vi "HeartBeatDetectRealTime1Valsalva.vi"() -> ()   [LabVIEW 2014, in "Phonocardiography.lvlib"]
uses:
  Phonocardiography.lvlib
  <vilib>/sound2/lvsound2.llb/Sampling Mode.ctl
  <vilib>/sound2/lvsound2.llb/Sound Data Format.ctl
  <vilib>/Platform/TimedLoop/XDataNode/timing_clust.ctl
  <vilib>/Platform/TimedLoop/XDataNode/nitl_modes.ctl
  <vilib>/Platform/TimedLoop/XDataNode/wakeup.ctl
  <vilib>/sound2/lvsound2.llb/Sound Input Read (DBL).vi
  <vilib>/Waveform/WDTOps.llb/WDT Get Waveform Time Array DBL.vi
  <vilib>/platform/TimedLoop/XDataNode/XDataNode.xnode
  <vilib>/Analysis/NI_AAL_SigProc.lvlib
  <vilib>/Platform/TimedLoop/XDataNode/XDNodeRunTimeDep.lvlib
  <vilib>/Analysis/NI_AALBase.lvlib
panel:
  in  "Exhale length [s]":dbl=6.0
  out "Inhale":bool
  in  "Init length [s]":dbl=6.0
  in  "Stop":bool
  in  "Window length [s]":dbl=0.95 min=0.0 max=50.0 step=0.05
  in  "Save to":path=path "C:/Users/Tamas/Documents/Projektek/Magzati szívhang/Felvételek cikkhez/breath_2.wav"
  in  "Samples per\nLoop":i32=8192
  in  "Device ID":u32
  in  "Stop & Save":bool
  out "Heart rate":T1(graph)=[{"X [s]"=[1.3810454402648886, 2.1451014620294155, 2.834039083155719, 3.5082652214542707, 4.267812415306186, 5.283414824587101, 6.333745411581, 7.352497923020055, 8.340778421797614, 9.286742620731337, 10.168091052124844, 11.008353434253126, 11.766188704199886, 12.459857993882613, 13.160303085008367, 13.937005708439617, 14.916256103906665, 15.990392513713077, 17.026184719534893, 18.025566635405323, 18.97826048371807, 19.895876149785295, 20.77148344893412, 21.58219271330085, 22.317733593752568, 23.026818175608778, 23.777685137270783, 24.65158299378833, 25.66356423384652, 26.69873921266114, 27.752698470400272, 28.772013707647154, 29.742896014934153, 30.650118429443005, 31.470679114349547, 32.19628263399749, 32.89445774972244, 33.66604914709347, 34.53537473985873, 35.51529057371639, 36.547147137879335, 37.577860857157, 38.55405439667892, 39.45290864114518, 40.309631377497524, 41.11504533403093, 41.84509526458157, 42.525847910413134, 43.23209659612331, 44.06765071982923, 44.96984707542182, 45.947480314447624, 46.920868322812716, 47.837254170634964, 48.70405945356165, 49.504490542408455, 50.220753683982565, 50.91447600262699, 51.59735912079533, 52.30215614364477, 53.04693497173172, 53.877926380484645, 54.78308482581491, 55.72546544156374, 56.671367006023424, 57.591099754403, 58.475088172441076, 59.293003678840876, 60.046376669503445, 60.79669511272331, 61.52442997106812, 62.25025157154459, 63.012813377936496, 63.8271252008184, 64.76642444301858, 65.69495143489829, 66.61622522259673, 67.50133872767269, 68.32457083017923, 69.10155513831889, 69.84249179812262, 70.6376427542073, 71.43050342495626, 72.15710097862082, 72.869491186341, 73.59336989453159, 74.37313142224703, 75.27019769563682, 76.15832609501031, 77.03212650593542, 77.90552889801594, 78.77465743537506, 79.62075706292664, 80.45163850714349, 81.1982417174044, 81.8712051082844, 82.52583434169513, 83.20775444122651, 84.0216953422601, 84.87335076971661, 85.79249037575387, 86.73069894059917, 87.64715321189007, 88.53326116001448, 89.36559786895394, 90.15065708658227, 90.87383450984113, 91.54145150844631, 92.21301976186118, 92.94571852487775, 93.7510641244373, 94.64661578749286, 95.54741044208302, 96.5225663414621, 97.52177353097777, 98.48706973490316, 99.44226945816028, 100.37012376206445, 101.23467811616628, 101.98654166591145, 102.67171477694043, 103.36534981417746, 104.11316781035048, 104.97669498014312, 105.91515824719292, 106.88001332870756, 107.80736044827695, 108.70537037239123, 109.55381284940862, 110.3611828413852, 111.11257513889484, 111.80992721929452, 112.53266423876909, 113.371875704155, 114.23971177605979, 115.15354851469199, 116.12435502467058, 117.11297189324033, 118.07091168953183, 118.96774342793292, 119.82781735444664, 120.67884494275361, 121.4691175113743, 122.20823957402418], "Heart Rate [BPM]"=[68.40647655058463, 78.5282731774494, 87.09061337354396, 88.99091357005743, 78.99443311181248, 59.07823716416964, 57.12487167656724, 58.89556033118001, 60.71150859924507, 63.42734753348079, 68.07750245284211, 71.40626699011246, 79.17287882921464, 86.49654942550936, 85.65981939222115, 77.24964251432185, 61.27135641480476, 55.85882710261502, 57.926676473101054, 60.03710798362997, 62.97930873203597, 65.3868522724245, 68.52386915724182, 74.00926896631427, 81.5726244381578, 84.61613964716969, 79.90763086338636, 68.65790956290691, 59.28963663056629, 57.96121547364511, 56.928196758484795, 58.863046295723876, 61.799457616713596, 66.13593209387643, 73.12073452170533, 82.68978633002146, 85.93832499701593, 77.76136463474401, 69.01901945523561, 61.229748440533335, 58.14761671712856, 58.21209020294084, 61.46322175967706, 66.75164563040832, 70.03432668947367, 74.49585335998746, 82.1861594517855, 88.13774043684857, 84.95591031035492, 71.80863369315091, 66.50436972846161, 61.372708705965145, 61.640373093126925, 65.4746034572527, 69.21969810499517, 74.95960718672598, 83.76809655197358, 86.48993752607461, 87.86276656089348, 85.13089308667135, 80.56082925197656, 72.20291253075968, 66.28673721108329, 63.66854219759496, 63.43154748271637, 65.2363418674726, 67.87419243926723, 73.35721053156293, 79.64182515652938, 79.9660471392918, 82.44761029651161, 82.66494130322529, 78.68214680707973, 73.68184805134712, 63.87740701191062, 64.61847692605704, 65.12721929264292, 67.78791607619927, 72.88345512439918, 77.22163674535267, 80.97858191534635, 75.45737012684927, 75.67533895119668, 82.57666117562985, 84.22350468855369, 82.8868142150163, 76.94660209229534, 66.88469044017728, 67.55779912265608, 68.66556624352756, 68.69685787907532, 69.03466797018595, 70.91363480873557, 72.21246835829115, 80.363972690436, 89.15789597639342, 91.65493524844545, 87.98684778646678, 73.71542568239107, 70.45102757014268, 65.27844040872237, 63.951665171478695, 65.46971505243243, 67.71184044449664, 72.0862114521537, 76.42735560925004, 82.96719182634531, 89.87188781195628, 89.34311545387331, 81.88904230297295, 74.50217649765996, 66.99780981399154, 66.60785529116924, 61.528623308544454, 60.047606371890396, 62.1570868672322, 62.81408855040989, 64.66532487647643, 69.39991651806916, 79.80171404816222, 87.56911068779753, 86.50082071834085, 80.23342619066719, 69.48246922492017, 63.93430846645616, 62.18550448613611, 64.70069161142244, 66.81440637661001, 70.71781720656415, 74.31537039555965, 79.85176345147495, 86.03975192217317, 83.01774834174188, 71.49568669490081, 69.13748107785794, 65.6572421128593, 61.80428271059227, 60.69085194429577, 62.6344163091249, 66.9021817927302, 69.7614450925258, 70.5030022814692, 75.92317180478933, 81.17739008478434]}, {"X [s]"=array[1351680 elements], "Heart Rate [BPM]"=array[1351680 elements]}]
  out "pNN50 [%]":dbl=22.377622377622377 format="%0.2f"
  out "rMSSD  [ms]":dbl=63.69905592461299 format="%0.2f"
  out "sdRR [ms]":dbl=107.76134947819452 format="%0.2f"
  out "Mean RR [ms]":dbl=845.1687782348819 format="%0.2f"
  out "Mean heart rate [BPM]":dbl=70.99173744362493
  out "Peaks":cluster{dbl[], "Amplitudes":dbl[]}[](graph)=[{array[1351680 elements], "Amplitudes"=array[1351680 elements]}, {[0.503935508201194, 1.3810454402648886, 2.1451014620294155, 2.834039083155719, 3.5082652214542707, 4.267812415306186, 5.283414824587101, 6.333745411581, 7.352497923020055, 8.340778421797614, 9.286742620731337, 10.168091052124844, 11.008353434253126, 11.766188704199886, 12.459857993882613, 13.160303085008367, 13.937005708439617, 14.916256103906665, 15.990392513713077, 17.026184719534893, 18.025566635405323, 18.97826048371807, 19.895876149785295, 20.77148344893412, 21.58219271330085, 22.317733593752568, 23.026818175608778, 23.777685137270783, 24.65158299378833, 25.66356423384652, 26.69873921266114, 27.752698470400272, 28.772013707647154, 29.742896014934153, 30.650118429443005, 31.470679114349547, 32.19628263399749, 32.89445774972244, 33.66604914709347, 34.53537473985873, 35.51529057371639, 36.547147137879335, 37.577860857157, 38.55405439667892, 39.45290864114518, 40.309631377497524, 41.11504533403093, 41.84509526458157, 42.525847910413134, 43.23209659612331, 44.06765071982923, 44.96984707542182, 45.947480314447624, 46.920868322812716, 47.837254170634964, 48.70405945356165, 49.504490542408455, 50.220753683982565, 50.91447600262699, 51.59735912079533, 52.30215614364477, 53.04693497173172, 53.877926380484645, 54.78308482581491, 55.72546544156374, 56.671367006023424, 57.591099754403, 58.475088172441076, 59.293003678840876, 60.046376669503445, 60.79669511272331, 61.52442997106812, 62.25025157154459, 63.012813377936496, 63.8271252008184, 64.76642444301858, 65.69495143489829, 66.61622522259673, 67.50133872767269, 68.32457083017923, 69.10155513831889, 69.84249179812262, 70.6376427542073, 71.43050342495626, 72.15710097862082, 72.869491186341, 73.59336989453159, 74.37313142224703, 75.27019769563682, 76.15832609501031, 77.03212650593542, 77.90552889801594, 78.77465743537506, 79.62075706292664, 80.45163850714349, 81.1982417174044, 81.8712051082844, 82.52583434169513, 83.20775444122651, 84.0216953422601, 84.87335076971661, 85.79249037575387, 86.73069894059917, 87.64715321189007, 88.53326116001448, 89.36559786895394, 90.15065708658227, 90.87383450984113, 91.54145150844631, 92.21301976186118, 92.94571852487775, 93.7510641244373, 94.64661578749286, 95.54741044208302, 96.5225663414621, 97.52177353097777, 98.48706973490316, 99.44226945816028, 100.37012376206445, 101.23467811616628, 101.98654166591145, 102.67171477694043, 103.36534981417746, 104.11316781035048, 104.97669498014312, 105.91515824719292, 106.88001332870756, 107.80736044827695, 108.70537037239123, 109.55381284940862, 110.3611828413852, 111.11257513889484, 111.80992721929452, 112.53266423876909, 113.371875704155, 114.23971177605979, 115.15354851469199, 116.12435502467058, 117.11297189324033, 118.07091168953183, 118.96774342793292, 119.82781735444664, 120.67884494275361, 121.4691175113743, 122.20823957402418], "Amplitudes"=[0.25504343516715083, 0.26274397594688526, 0.22978339915261922, 0.2925323075507681, 0.2597312409018822, 0.3127614804590793, 0.28443490759254775, 0.27205766410251664, 0.3588946349377459, 0.30343314882440386, 0.31376920698615113, 0.322137223701114, 0.2810882365066251, 0.27506508906369076, 0.30417811837100495, 0.3072988366388709, 0.3531073610883032, 0.35795320527487806, 0.3052941945137585, 0.31661824578621095, 0.30039393277341386, 0.2773968250538757, 0.26402954583415333, 0.2935481885611599, 0.25451231358440163, 0.2579234365250457, 0.2912559504206825, 0.34990378193234895, 0.3496948360558424, 0.3567944199797841, 0.2880780844317378, 0.35024483155485536, 0.3079129335486051, 0.277514077912824, 0.2682372059613101, 0.2454065764686712, 0.2751967493505104, 0.3148522910083886, 0.3609840914449288, 0.34310706318641965, 0.34544899314122623, 0.31836698955515097, 0.336588819016225, 0.28998981599808693, 0.2746642353091651, 0.2930369693584984, 0.25632591284717665, 0.280905641938724, 0.3034019557433223, 0.33740367919858355, 0.37820946496973956, 0.3762582381068588, 0.36079169943917255, 0.351891937904827, 0.344543955968987, 0.2954466736592642, 0.27290683472441535, 0.29208699683305334, 0.2467246065441302, 0.2734435147341604, 0.33840264581773954, 0.3758157913766263, 0.41797426044197444, 0.3987311037373865, 0.3522034833047552, 0.34301282991047993, 0.32333772821889795, 0.3275101426458208, 0.3252370381018068, 0.3080495835018164, 0.28518800214775536, 0.29187945059952636, 0.3239309006163301, 0.35145605790417883, 0.366627975838492, 0.38681638063755935, 0.34644556204490734, 0.3088510834350089, 0.32315301230300625, 0.3278101986496201, 0.32359254170972934, 0.3128436889466553, 0.2911982399566819, 0.2702401508417269, 0.2837937098744517, 0.3561313602989965, 0.366025748700734, 0.3745793451140769, 0.4013420308747677, 0.36342594915295023, 0.36429667870898036, 0.3453740341837724, 0.3227150331693566, 0.33087300820788496, 0.2916365225649727, 0.28274935921864214, 0.3371922556538561, 0.3551343026648233, 0.3794991663138844, 0.4215358387379555, 0.3909484882661073, 0.4020134751412901, 0.35311185806805917, 0.3574730866113045, 0.3390535985260016, 0.33676288810446586, 0.3371554462632124, 0.33345259263923643, 0.23478686751538175, 0.2900521506472944, 0.3525789301399259, 0.30563158999499523, 0.36031172340677264, 0.3511990527765965, 0.33790226481271984, 0.30568150243560205, 0.312684134983506, 0.2873402577165768, 0.3311034578064147, 0.27303866289452006, 0.27201102337444394, 0.31721392757280864, 0.3481193098154417, 0.3523428926132475, 0.33526402963698154, 0.34410895558312143, 0.316476698827496, 0.32363953395355666, 0.32656456873670986, 0.3402988608986353, 0.3162552341260466, 0.3030898408720127, 0.26323398331948644, 0.29143756579258123, 0.35945221685073125, 0.3460112044221787, 0.3371709234039179, 0.3309440762172199, 0.3246586520069406, 0.3857515596346559, 0.3517691325334278, 0.32204782859753883, 0.29833629675859463, 0.26478829805647797, 0.2888316659968011]}]
  in  "Threshold mult":dbl=0.8 min=-1.0 max=1.0 step=0.05
  in  "width (threshold)":i32=200
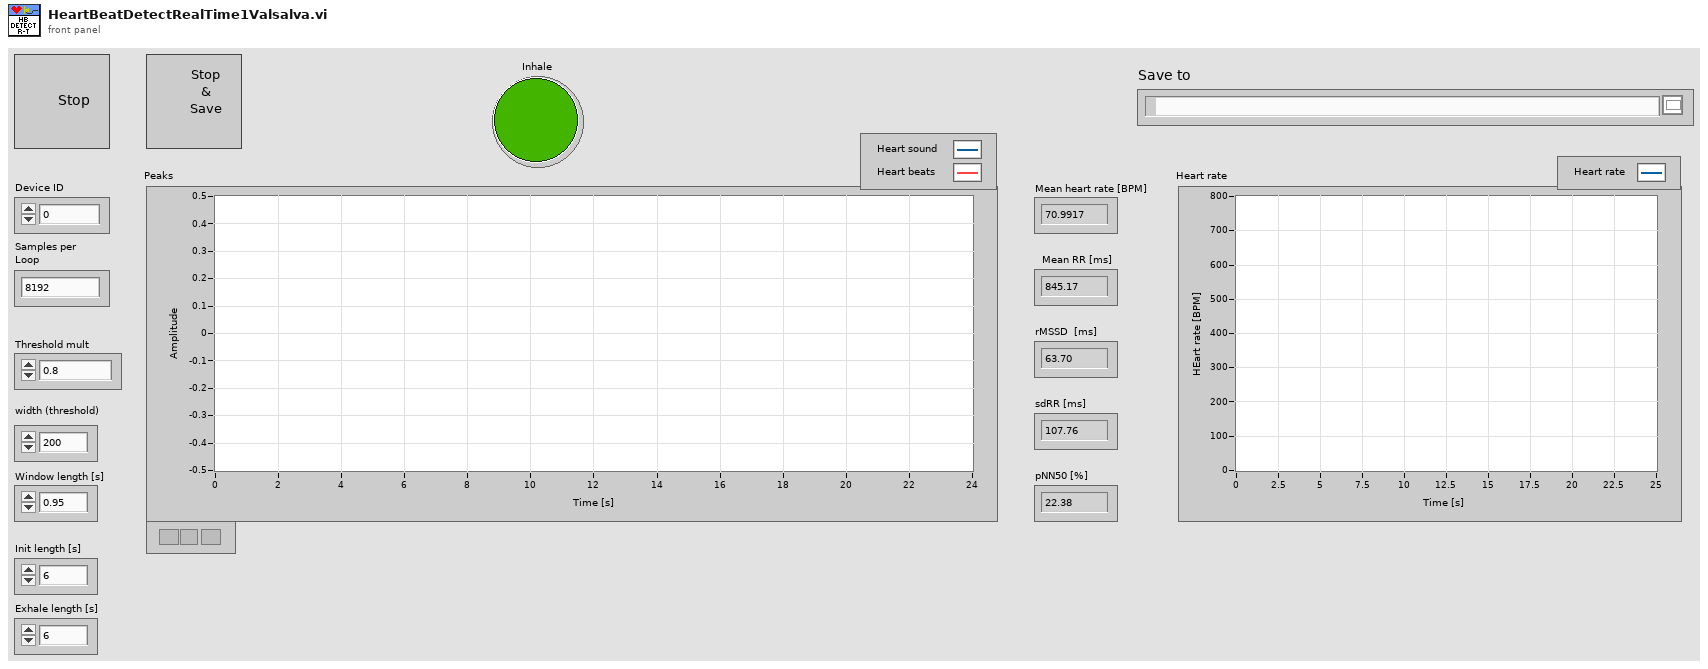
[diagram p1: front panel]
types:
  T1 = cluster{"X [s]":dbl[], "Heart Rate [BPM]":dbl[]}[]
  T2 = typedef "Sound Data Format.ctl" = cluster{"sample rate (S/s)":dbl, "number of channels":i32, "bits per sample":i32}
  T3 = typedef "Sampling Mode.ctl" = i32
  T4 = typedef "XDNodeRunTimeDep.lvlib/timing_clust.ctl" = cluster{"Expected End [f-1]":u64, "Actual End [f-1]":u64, "Finished Late? [f-1]":bool, "Expected End [i-1]":u64, "Actual End [i-1]":u64, "Finished Late? [i-1]":bool, "Expected Start [i]":u64, "Actual Start [i]":u64, "Expected Start [f]":u64, "Actual Start [f]":u64, "Source Name":string, "Structure Name":string, "Period":i64, "Deadline":i64, "Offset":i64, "Start":i64, "Priority":i32, "Timeout":i32, "Mode":T5, "Wakeup Reason":T6, "Error":errorcluster, "Source Type":string, "Secondary Source Type":string, "Global End Time":u64, "Global Start Time":u64, "Frame Duration":u64, "Iteration Duration":u64, "Assigned CPU":i32, "I/O Scan Engine Mode":u32}
  T5 = typedef "XDNodeRunTimeDep.lvlib/nitl_modes.ctl" = enum32{"No Change", "Process missed periods, maintain original phase", "Discard missed periods, maintain original phase", "Process missed periods, ignore original phase", "Discard missed periods, ignore original phase"}
  T6 = typedef "XDNodeRunTimeDep.lvlib/wakeup.ctl" = enum32{"Normal", "Aborted", "Asynchronous wakeup", "Timing source error", "Timed loop error", "Timeout"}
  T7 = typedef "Sound Input Task ID.ctl" = u32
  T8 = typedef "LVCursorListTypeDef.ctl" = cluster{"Name":string, "Color":u32, "Style":u8, "Point Style":u8, "Name Visible":bool, "Allow Drag":bool, "Cursor Mode":u32, "Plot":i32, "Index":i32, "Position":cluster{"X":dbl, "Y":dbl}, "X Scale":u32, "Y Scale":u32, "Watch Plots":i32[], "Watch All Plots":bool, "Plot Area":i32, "Label Offset":cluster{"X":dbl, "Y":dbl}}[]
  T9 = cluster{"Name":string, "Color":u32, "Style":u8, "Point Style":u8, "Name Visible":bool, "Allow Drag":bool, "Cursor Mode":u32, "Plot":i32, "Index":i32, "Position":cluster{"X":dbl, "Y":dbl}, "X Scale":u32, "Y Scale":u32, "Watch Plots":i32[], "Watch All Plots":bool, "Plot Area":i32, "Label Offset":cluster{"X":dbl, "Y":dbl}}
  T10 = cluster{"Name":string, "Color":u32, "Style":u8, "Point Style":u8, "Name Visible":bool, "Allow Drag":bool, "Cursor Mode":u32, "Plot":i32, "Index":i32, "Position":cluster{"X":dbl, "Y":dbl}, "X Scale":u32, "Y Scale":u32, "Watch Plots":i32[], "Watch All Plots":bool, "Plot Area":i32, "Label Offset":cluster{"X":dbl, "Y":dbl}}[]
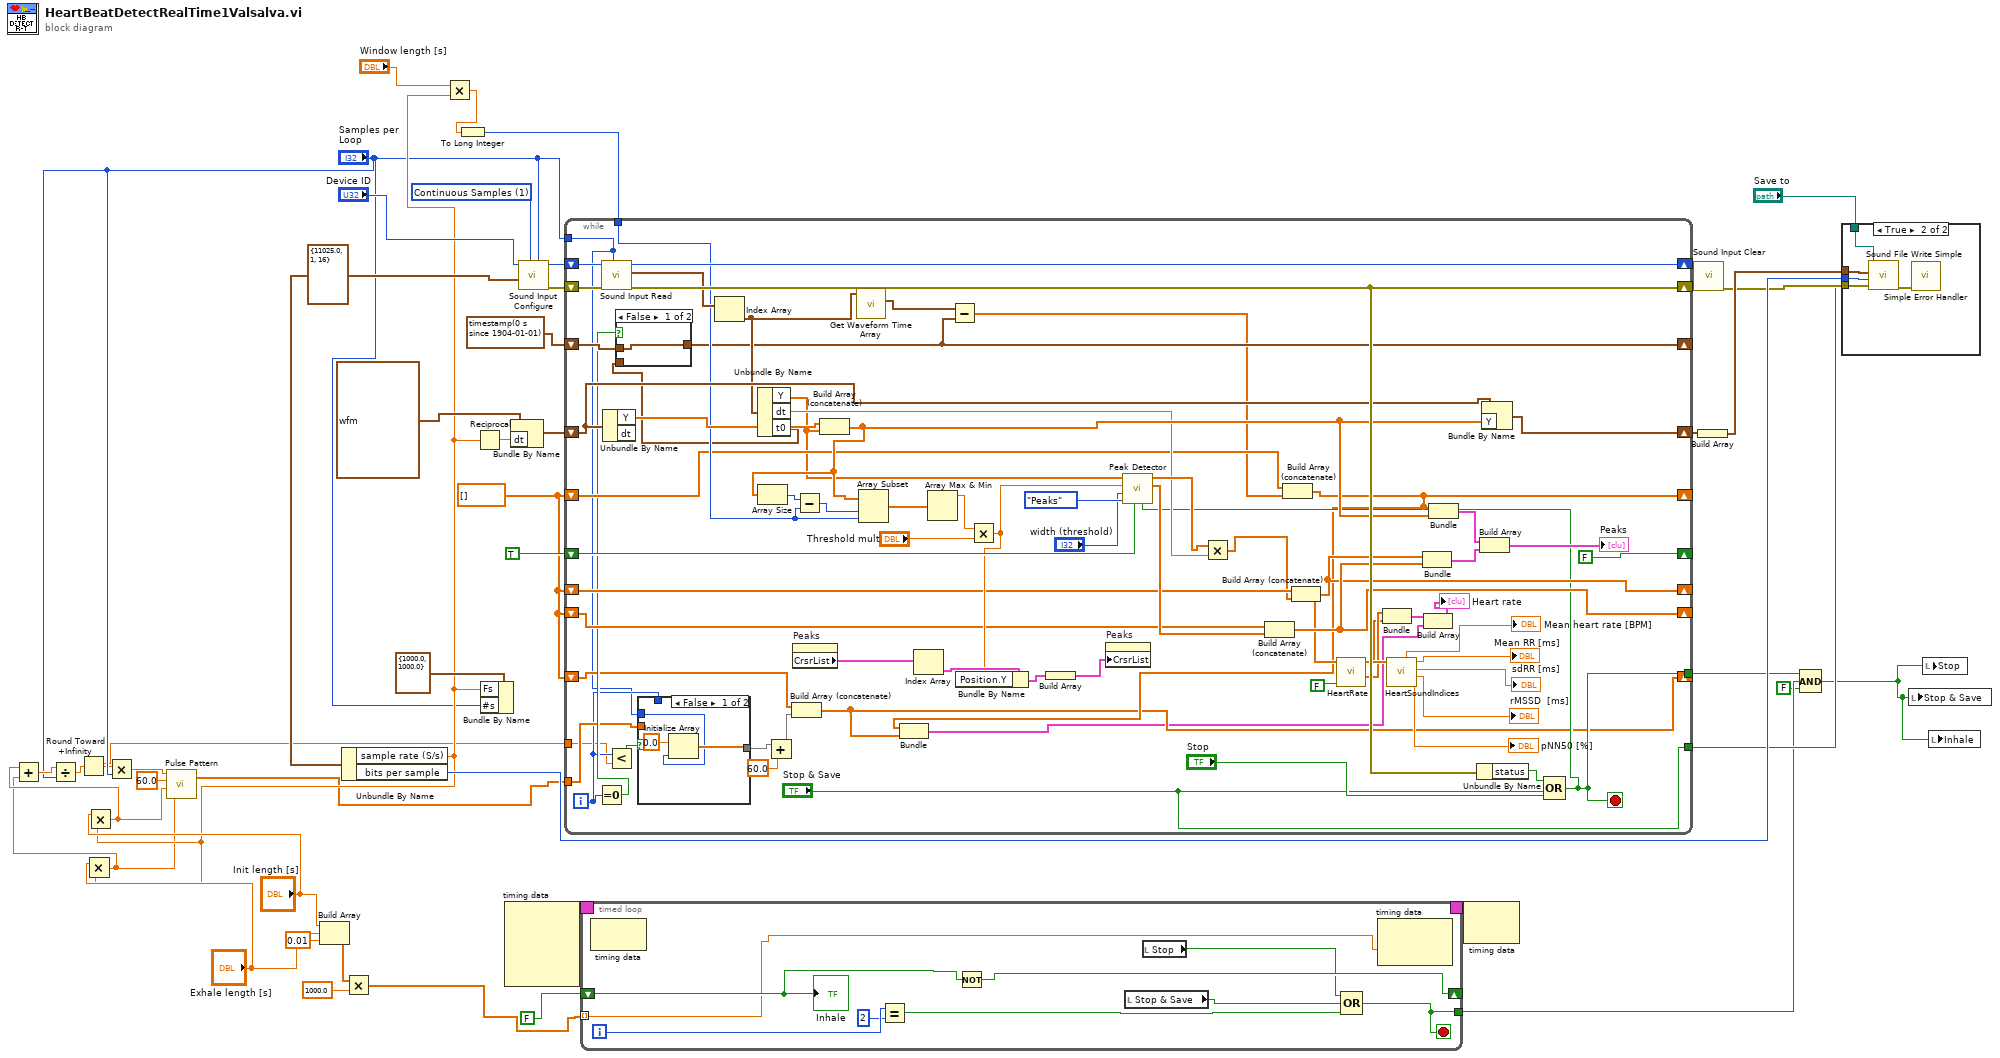
[diagram p0: block diagram]
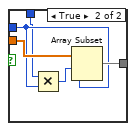
[diagram p3: hidden frame]
diagram:
  w18 = dbl[] []
  w40 = T2 {"sample rate (S/s)"=11025.0, "number of channels"=1, "bits per sample"=16} ("Sound Format")
  w46 = T3 1 items=["Finite Samples", "Continuous Samples"] ("sample mode")
  n1 = Build Array("Init length [s]", "Exhale length [s]", 0.01 ("element")) -> (w16:dbl[])
  n2 = Unbundle By Name(w40) -> ("sample rate (S/s)"=w10:dbl, "bits per sample"=w38:i32)
  n3 = Multiply(x="Exhale length [s]", y=w10) -> (x*y=w7:dbl)
  n4 = Multiply(x="Init length [s]", y=w10) -> (x*y=w8:dbl)
  n5 = Add(x=w8, y=w7) -> (x+y=w6:dbl)
  n6 = Divide(x=w6, y="Samples per\nLoop") -> (x/y=w5:dbl)
  n7 = Round Toward +Infinity(x=w5) -> (ceil(x): smallest int >= x=w1:dbl)
  n8 = Multiply(x=w1, y="Samples per\nLoop") -> (x*y=w3:dbl)
  n9 = call <vilib>:"Pulse Pattern.vi"("width"=w7, "delay"=w8, "amplitude"=60.0, "samples"=w3) -> ("Pulse Pattern"=w2:dbl[])  [unwired: 1 out]
  n10 = Multiply(x=w16, y=1000.0) -> (x*y=w15:dbl[])
  n11 = Multiply(x="Window length [s]", y=w10) -> (x*y=w30:dbl)
  n12 = To Long Integer(number=w30) -> (32bit integer=w29:i32)
  n13 = Reciprocal(x=w10) -> (1/x=w35:dbl)
  n14 = Bundle By Name(cluster=cluster{"Fs":dbl, "#s":dbl} {"Fs"=1000.0, "#s"=1000.0} ("sampling info"), "Fs"=w10, "#s"="Samples per\nLoop") -> ()  [unwired: 1 out]
  n15 = node-c288() -> (w25:T4)  [unwired: 4 in]
  n16 = Bundle By Name(cluster=waveform(dbl) {"t0"=timestamp(0 s since 1904-01-01), "dt"=1.0, "Y"=[]} ("element"), "dt"=w35) -> (w34:waveform(dbl))
  n17 = call <vilib>:"Sound Input Configure.vi"("number of samples/ch"="Samples per\nLoop", "sample mode"=w46, "sound format"=w40, "device ID"="Device ID") -> ("error out"=w42:errorcluster, "task ID"=w43:T7)  [unwired: 6 in]
  n18 = while {
    tunnel: "Samples per\nLoop" -> [w47]
    shift-right: [w115] -> w44
    shift-left: w43 -> [w116]
    shift-right: [w114] -> w45
    shift-left: w42 -> [w117]
    shift-right: [w110] -> w37
    shift-left: w34 -> [w111]
    tunnel: w29 -> [w107]
    shift-right: [FALSE] -> _
    shift-left: TRUE -> [w102]
    shift-right: [w59] -> _
    shift-left: w18 -> [w76]
    shift-right: [w69] -> _
    shift-left: w18 -> [w78]
    shift-right: [w77] -> _
    shift-left: w18 -> [w79]
    shift-right: [w71] -> _
    shift-left: timestamp(0 s since 1904-01-01) ("t0") -> [w74]
    tunnel: ["Stop & Save"] -> w26
    tunnel: [w62] -> w22
    shift-right: [w57] -> _
    shift-left: w18 -> [w58]
    tunnel: w2 -> [w53]
    tunnel: w1 -> [w51]
    i -> [w52]
    stop <- w62 stop-if-true
    n19 = Equal To 0?(x=w52) -> (x = 0?=w73:bool)
    n20 = call-poly <vilib>:"Sound Input Read.vi"("number of samples/ch"=w47, "error in (no error)"=w117, "task ID"=w116) -> ("error out"=w114:errorcluster, "data"=w113:waveform(dbl)[], "task ID out"=w115:T7)  [unwired: 6 in]
    n21 = Unbundle By Name(w111) -> ("Y"=w112:dbl[])  [unwired: 1 out]
    n22 = Less?(x=w52, y=w51) -> (x < y?=w54:bool)
    n23 = case shown="False" w54 {
      tunnel: w53 -> [_ w125]
      tunnel: w52 -> [_ w121]
      tunnel: w47 -> [w118 w122]
      tunnel: [w119 w123] -> w50
      frame False {
        n24 = Initialize Array(0.0 ("element"), w118) -> (w119:dbl[])
      }
      frame True {
        n25 = Multiply(x=w121, y=w122) -> (x*y=w124:i32)
        n26 = Array Subset(array=w125, index=w124, length=w122) -> (w123:dbl[])
      }
    }
    n27 = Index Array(array=w113) -> (element=w82:waveform(dbl))  [unwired: 1 in]
    n28 = Unbundle By Name(w82) -> ("Y"=w55:dbl[], "dt"=w81:dbl, "t0"=w72:timestamp)
    n29 = case shown="False" w73 {
      tunnel: w74 -> [w126 _]
      tunnel: w72 -> [_ w127]
      tunnel: [w126 w127] -> w71
      frame False {
      }
      frame True {
      }
    }
    n30 = Add(x=w50, y=60.0 ("amplitude")) -> (x+y=w48:dbl[])
    n31 = Build Array (concatenate)(w58, w48) -> (w57:dbl[])
    n32 = property on="Peaks" class="XYGraph (strict)"() -> ("CrsrList"=w97:T8)  [unwired: 2 in, 2 out]
    n33 = Build Array (concatenate)(w112, w55) -> (w83:dbl[])
    n34 = Array Size(array=w83) -> (size(s)=w108:i32)
    n35 = Subtract(x=w108, y=w107) -> (x-y=w106:i32)
    n36 = call-poly <vilib>:"Get Waveform Time Array.vi"("waveform in"=w82) -> ("X array"=w86:timestamp[])  [unwired: 9 in, 1 out]
    n37 = Array Subset(array=w83, index=w106, length=w107) -> (w105:dbl[])
    n38 = Index Array(array=w97) -> (element=w98:T9)  [unwired: 1 in]
    n39 = Array Max & Min(array=w105) -> (max value=w104:dbl)  [unwired: 3 out]
    n40 = Subtract(x=w86, y=w71) -> (x-y=w64:dbl[])
    n41 = Multiply(x=w104, y="Threshold mult") -> (x*y=w96:dbl)
    n42 = Bundle By Name(cluster=w98, "Position.Y"=w96) -> (w99:T9)
    n43 = Build Array(w99) -> (w100:T10)
    n44 = property on="Peaks" class="XYGraph (strict)"("CrsrList"=w100) -> ()  [unwired: 2 in, 2 out]
    n45 = Build Array (concatenate)(w76, w64) -> (w59:dbl[])
    n46 = Bundle(w59, w57) -> (w56:cluster{dbl[], dbl[]})  [unwired: 1 in]
    n47 = Bundle(w59, w83) -> (w87:cluster{dbl[], dbl[]})  [unwired: 1 in]
    n48 = Unbundle By Name(w114) -> ("status"=w109:bool)
    n49 = Bundle By Name(cluster=w111, "Y"=w83) -> (w110:waveform(dbl))
    n50 = Compound Arithmetic op=OR(w109, "Stop & Save", "Stop") -> (w62:bool)
    n51 = call <vilib>:"Peak Detector.vi"("end of data (T)"=w62, "initialize (T)"=w102, "peaks/valleys"=enum32{"Peaks", "Valleys"}."Peaks", "width"="width (threshold)", "threshold"=w96, "X"=w55) -> ("Amplitudes"=w80:dbl[], "Locations"=w84:dbl[])  [unwired: 1 in, 3 out]
    n52 = Multiply(x=w84, y=w81) -> (x*y=w63:dbl[])
    n53 = Build Array (concatenate)(w79, w80) -> (w77:dbl[])
    n54 = Build Array (concatenate)(w78, w63) -> (w69:dbl[])
    n55 = call "HeartRate.vi"("Remove Ectopic?"=FALSE, "Peaks X in"=w69) -> ("X [s]"=w89:dbl[], "RR intervals [ms]"=w90:dbl[], "Heart Rate [BPM]"=w88:dbl[])  [unwired: 7 in]
    n56 = Bundle("X [s]"=w89, "Heart Rate [BPM]"=w88) -> (w61:cluster{"X [s]":dbl[], "Heart Rate [BPM]":dbl[]})  [unwired: 1 in]
    n57 = call "HeartSoundIndices.vi"("RR intervals [ms]"=w90) -> ("pNN50 [%]"=→"pNN50 [%]":dbl, "rMSSD  [ms]"=→"rMSSD  [ms]":dbl, "sdRR [ms]"=→"sdRR [ms]":dbl, "Mean RR [ms]"=→"Mean RR [ms]":dbl, "Mean heart rate [BPM]"=→"Mean heart rate [BPM]":dbl)  [unwired: 6 in]
    n58 = Bundle(w69, w77) -> (w70:cluster{dbl[], dbl[]})  [unwired: 1 in]
    n59 = Build Array(w61, w56) -> (→"Heart rate":T1)
    n60 = Build Array(w87, w70) -> (→"Peaks":cluster{dbl[], dbl[]}[])
  }
  n61 = timed-loop {
    timing: w25 -> [_]
    timing-out: [_] -> w24
    shift-right: [w135] -> _
    shift-left: FALSE -> [w136]
    tunnel: [w132] -> w21
    tunnel: w15 -> [w128] mode=indexing
    i -> [w131]
    stop <- w132 stop-if-true
    n62 = node-c288() -> ()  [unwired: 1 in, 1 out]
    n63 = Equal?(x=w131, y=2) -> (x = y?=w129:bool)
    n64 = Not(x=w136) -> (.not. x?=w135:bool)
    n65 = local read "Stop & Save"() -> (w133:bool)
    n66 = local read "Stop"() -> (w134:bool)
    n67 = Compound Arithmetic op=OR(w134, w133, w129) -> (w132:bool)
    n68 = node-c288(w128) -> ()  [unwired: 1 in, 1 out]
    "Inhale" <- w136
  }
  n69 = node-c288(w24) -> ()  [unwired: 1 out]
  n70 = call <vilib>:"Sound Input Clear.vi"("error in (no error)"=w45, "task ID"=w44) -> ("error out"=w32:errorcluster)  [unwired: 9 in]
  n71 = Build Array(w37) -> (w39:waveform(dbl)[])
  n72 = Compound Arithmetic op=AND(w22, w21, FALSE ("value")) -> (w13:bool)
  n73 = case shown="True" w26 {
    tunnel: w39 -> [_ w145]
    tunnel: w38 -> [_ w144]
    tunnel: "Save to" -> [_ w142]
    tunnel: w32 -> [_ w141]
    frame False {
    }
    frame True {
      n74 = call <vilib>:"Sound File Write Simple.vi"("error in (no error)"=w141, "bits per sample"=w144, "data"=w145, "path"=w142) -> ("error out"=w143:errorcluster)  [unwired: 6 in, 1 out]
      n75 = call <vilib>:"Simple Error Handler.vi"("error in (no error)"=w143) -> ()  [unwired: 4 in, 5 out]
    }
  }
  n76 = local write "Stop & Save"(w13) -> ()
  n77 = local write "Stop"(w13) -> ()
  n78 = local write "Inhale"(w13) -> ()
